vi "HFRR ADV v038.vi"() -> ()   [LabVIEW 2025] (continued)
        n1305 = case shown="True" w1608 {
          selector: w1608 -> [_ w1614]
          frame False {
          }
          frame True {
            n1306 = Not(x=w1614) -> (.not. x?=w1613:bool)
            n1307 = local write "CAMERA ROI MIN TEMP"(w1613) -> ()
            n1308 = call "IMAGE ANALYSIS.vi"("Enum"=POST_ANALYSIS_ENUM."MINIMIZE UI") -> ()  [unwired: 9 in, 2 out]
          }
        }
      }
      frame "Mooha" {
        n1309 = local read "LIVE FEED MIN TEMP"() -> (w1620:bool)
        n1310 = local write "LIVE FEED MAX TEMP"(TRUE ("LIVE FEED MAX TEMP")) -> ()
        n1311 = local read "CAMERA ROI MIN TEMP"() -> (w1618:bool)
        n1312 = case shown="True" w1620 {
          selector: w1620 -> [_ w1627]
          frame False {
          }
          frame True {
            n1313 = Not(x=w1627) -> (.not. x?=w1626:bool)
            n1314 = local write "LIVE FEED MIN TEMP"(w1626) -> ()
            n1315 = call "CAMERA LIVE FEED FGV.vi"("Enum - Menu"=CAMERA_LIVE_FEED_ENUM."CAMERA MINIMIZE") -> ()  [unwired: 9 in, 2 out]
          }
        }
        n1316 = local write "CAMERA ROI MAX TEMP"(TRUE ("CAMERA ROI MAX TEMP")) -> ()
        n1317 = case shown="True" w1618 {
          selector: w1618 -> [_ w1624]
          frame False {
          }
          frame True {
            n1318 = Not(x=w1624) -> (.not. x?=w1623:bool)
            n1319 = local write "CAMERA ROI MIN TEMP"(w1623) -> ()
            n1320 = call "IMAGE ANALYSIS.vi"("Enum"=POST_ANALYSIS_ENUM."MINIMIZE UI") -> ()  [unwired: 9 in, 2 out]
          }
        }
      }
    }
    n1321 = local read "Auto Start Test"() -> (w1365:bool)
    n1322 = case shown="True" "sign in temp" {
      frame False {
      }
      frame True {
        w1400 = 1 ("y")
        n1323 = local read "USERNAME"() -> (w1406:string)
        n1324 = local read "USER ID"() -> (w1403:string)
        n1325 = call <vilib>:"Trim Whitespace.vi"("string"=w1406) -> ("trimmed string"=w1405:string)  [unwired: 1 in]
        n1326 = call <vilib>:"Trim Whitespace.vi"("string"=w1403) -> ("trimmed string"=w1404:string)  [unwired: 1 in]
        n1327 = String Length(string=w1405) -> (length=w1402:i32)
        n1328 = String Length(string=w1404) -> (length=w1401:i32)
        n1329 = Greater?(x=w1402, y=w1400) -> (0:w1399:bool)
        n1330 = Greater?(x=w1401, y=w1400) -> (0:w1398:bool)
        n1331 = And(x=w1399, y=w1398) -> (x .and. y?=w1397:bool)
        n1332 = case shown="True" w1397 {
          frame False {
            n1333 = property on="Sign In" class="Bool (strict)"("DisabledEnum"=T19."Disabled" ("Disabled")) -> ()  [unwired: 2 in, 2 out]
          }
          frame True {
            n1334 = property on="Sign In" class="Bool (strict)"("DisabledEnum"=T19."Enabled" ("Disabled")) -> ()  [unwired: 2 in, 2 out]
          }
        }
      }
    }
    n1335 = local read "Air Temperature"() -> (w1382:bool)
    n1336 = local read "Coefficient Of Friction"() -> (w1383:bool)
    n1337 = case shown="False" w1365 {
      frame False {
        n1338 = local read "Auto stop temp"() -> (w1394:bool)
        n1339 = case shown="True" w1394 {
          frame False {
          }
          frame True {
            n1340 = local write "Auto Start Temp"(FALSE ("Auto Start Temp")) -> ()
          }
        }
      }
      frame True {
        "Auto stop temp" <- TRUE ("Auto stop temp")
      }
    }
    n1341 = local read "Humidity"() -> (w1381:bool)
    n1342 = case shown="\"HOME\"" w1391 {
      frame "HOME" {
        n1343 = local write "main tab sub"(enum32{"Page 1", "Page 2"}."Page 1" ("main tab sub")) -> ()
      }
      frame Default {
        n1344 = local write "main tab sub"(enum32{"Page 1", "Page 2"}."Page 2" ("main tab sub")) -> ()
      }
    }
    n1345 = case shown="True" w1390 {
      selector: w1390 -> [_ w1742]
      frame False {
      }
      frame True {
        n1346 = Not(x=w1742) -> (.not. x?=w1741:bool)
        n1347 = local write "Sign In"(w1741) -> ()
        n1348 = local write "Main Dashboard Buttons"(T26."Test Setup" ("Main Dashboard Buttons")) -> ()
      }
    }
    n1349 = case shown="\"Numeric Display\", Default" "Num/Graph" {
      frame "Numeric Display", Default {
        n1350 = property on="Single/Multiple" class="RadioBtnsControl (strict)"("Visible"=FALSE) -> ()  [unwired: 2 in, 2 out]
        n1351 = property on="Single - Graph" class="Ring (strict)"("Visible"=FALSE) -> ()  [unwired: 2 in, 2 out]
        n1352 = local write "Main Tab Display"(T4."Dashboard 1" ("Main Tab Display")) -> ()
      }
      frame "Graph Display" {
        n1353 = property on="Single/Multiple" class="RadioBtnsControl (strict)"("Visible"=TRUE) -> ()  [unwired: 2 in, 2 out]
        n1354 = case shown="\"Multiple\"" "Single/Multiple" {
          frame "Single ", Default {
            n1355 = property on="Single - Graph" class="Ring (strict)"("Visible"=TRUE) -> ()  [unwired: 2 in, 2 out]
            n1356 = local write "Main Tab Display"(T4."Dashboard 3" ("Main Tab Display")) -> ()
          }
          frame "Multiple" {
            n1357 = property on="Single - Graph" class="Ring (strict)"("Visible"=FALSE) -> ()  [unwired: 2 in, 2 out]
            n1358 = local write "Main Tab Display"(T4."Dashboard 2" ("Main Tab Display")) -> ()
          }
        }
      }
    }
    n1359 = local read "Stroke"() -> (w1380:bool)
    n1360 = local read "USERNAME"() -> (w1385:string)
    n1361 = case shown="True" w1383 {
      selector: w1383 -> [_ w1667]
      frame False {
      }
      frame True {
        n1362 = Not(x=w1667) -> (.not. x?=w1666:bool)
        n1363 = local write "Coefficient Of Friction"(w1666) -> ()
        n1364 = local write "Tab Control 2"(T6."Coefficient Of Friction" ("Tab Control 2")) -> ()
      }
    }
    n1365 = case shown="True" w1382 {
      selector: w1382 -> [_ w1664]
      frame False {
      }
      frame True {
        n1366 = Not(x=w1664) -> (.not. x?=w1662:bool)
        n1367 = local write "Air Temperature"(w1662) -> ()
        n1368 = local write "Tab Control 2"(T6."Air Temperature" ("Tab Control 2")) -> ()
      }
    }
    n1369 = case shown="True" w1380 {
      selector: w1380 -> [_ w1658]
      frame False {
      }
      frame True {
        n1370 = Not(x=w1658) -> (.not. x?=w1656:bool)
        n1371 = local write "Stroke"(w1656) -> ()
        n1372 = local write "Tab Control 2"(T6."Stroke" ("Tab Control 2")) -> ()
      }
    }
    n1373 = local write "tested by"(w1385) -> ()
    n1374 = case shown="True" w1381 {
      selector: w1381 -> [_ w1661]
      frame False {
      }
      frame True {
        n1375 = Not(x=w1661) -> (.not. x?=w1659:bool)
        n1376 = local write "Humidity"(w1659) -> ()
        n1377 = local write "Tab Control 2"(T6."Humidity" ("Tab Control 2")) -> ()
      }
    }
    n1378 = case shown="\"Calibration\"" "Main Dashboard Buttons" {
      tunnel: [T2."HOME" ("Main Tab") T2."Test Setup" ("Main Tab") T2."Acquire" ("Main Tab") T2."Adv Scar" ("Main Tab") T2."Adv Scar Report" ("Main Tab") T2."Compare Files" ("Main Tab") T2."Calibration" ("Main Tab") T2."About" ("Main Tab") T2."Advance" ("Main Tab")] -> w1364
      frame "Home", Default {
      }
      frame "Test Setup" {
      }
      frame "Dashboard" {
      }
      frame "Imaging" {
      }
      frame "Report" {
      }
      frame "Analysis" {
      }
      frame "Calibration" {
      }
      frame "About" {
      }
      frame "Advance" {
      }
    }
    n1379 = Wait (ms)(milliseconds to wait=u32 100) -> ()  [unwired: 1 out]
    n1380 = local read "Main Tab Display"() -> (w1384:T4)
    n1381 = local write "Main Tab"(w1364) -> ()
    n1382 = case shown="\"Dashboard 3\"" w1384 {
      frame "Dashboard 1", Default {
        n1383 = property on="Reset Graph" class="Bool (strict)"("Visible"=FALSE) -> ()  [unwired: 2 in, 2 out]
      }
      frame "Dashboard 2" {
        n1384 = property on="Reset Graph" class="Bool (strict)"("Visible"=TRUE) -> ()  [unwired: 2 in, 2 out]
      }
      frame "Dashboard 3" {
        n1385 = property on="Reset Graph" class="Bool (strict)"("Visible"=TRUE) -> ()  [unwired: 2 in, 2 out]
      }
    }
    n1386 = local read "SCAR MEASURMENT"() -> (w1372:enum32{"Auto Scar", "Manual Scar"})
    n1387 = local read "Humidity"() -> (w1386:bool)
    n1388 = local read "Cap Live Image"() -> (w1369:bool)
    n1389 = local read "Sample Temperature"() -> (w1379:bool)
    n1390 = local read "Air Temp vs Humidity"() -> (w1377:bool)
    n1391 = local read "Frequency"() -> (w1378:bool)
    n1392 = case shown="False" w1386 {
      frame False {
        n1393 = local write "Humidity On Command"(TRUE ("Humidity On Command")) -> ()
        n1394 = case shown="True" "Humidity Off Command" {
          selector: "Humidity Off Command" -> [_ w1674]
          frame False {
          }
          frame True {
            n1395 = stacked-sequence {
              frame #0 {
                n1396 = local read "WriteHumidity"() -> (w1676:string[])
                n1397 = Insert Into Array(array=w1676, new element="R;1" ("new element/subarray")) -> (w1675:string[])  [unwired: 1 in]
                n1398 = local write "WriteHumidity"(w1675) -> ()
              }
              frame #1 {
                n1399 = Wait (ms)(milliseconds to wait=u32 500) -> ()  [unwired: 1 out]
              }
              frame #2 {
                n1400 = local read "WriteHumidity"() -> (w1680:string[])
                n1401 = local read "EVENT LOG"() -> (w1684:string)
                n1402 = call "Event Log.vi"("Content"="Humidity Control Off" ("string"), "EVENT LOG"=w1684) -> ("EVENT LOG"=w1685:string)  [unwired: 8 in, 1 out]
                n1403 = local write "EVENT LOG"(w1685) -> ()
                n1404 = Insert Into Array(array=w1680, new element="R;1" ("new element/subarray")) -> (w1681:string[])  [unwired: 1 in]
                n1405 = local write "WriteHumidity"(w1681) -> ()
                n1406 = local write "Humidity"(TRUE ("Humidity")) -> ()
              }
            }
            n1407 = Not(x=w1674) -> (.not. x?=w1673:bool)
            n1408 = local write "Humidity Off Command"(w1673) -> ()
          }
        }
      }
      frame True {
        n1409 = local write "Humidity Off Command"(TRUE ("Humidity Off Command")) -> ()
        n1410 = case shown="False" "Humidity On Command" {
          selector: "Humidity On Command" -> [_ w1689]
          frame False {
          }
          frame True {
            n1411 = stacked-sequence {
              frame #0 {
                n1412 = local read "Set Rh"() -> (w1695:dbl)
                n1413 = local read "WriteHumidity"() -> (w1691:string[])
                n1414 = Number To Fractional String(number=w1695, precision (6)=i16 2) -> (F-format string=w1696:string)  [unwired: 2 in]
                n1415 = Concatenate Strings("M;" ("new element/subarray"), w1696) -> (w1694:string)
                n1416 = Insert Into Array(array=w1691, new element=w1694) -> (w1690:string[])  [unwired: 1 in]
                n1417 = local write "WriteHumidity"(w1690) -> ()
              }
              frame #1 {
                n1418 = Wait (ms)(milliseconds to wait=u32 500) -> ()  [unwired: 1 out]
              }
              frame #2 {
                n1419 = local read "WriteHumidity"() -> (w1699:string[])
                n1420 = local read "Set Rh"() -> (w1703:dbl)
                n1421 = Number To Fractional String(number=w1703, precision (6)=i16 2) -> (F-format string=w1704:string)  [unwired: 2 in]
                n1422 = Concatenate Strings("M;" ("new element/subarray"), w1704) -> (w1702:string)
                n1423 = Insert Into Array(array=w1699, new element=w1702) -> (w1698:string[])  [unwired: 1 in]
                n1424 = local write "WriteHumidity"(w1698) -> ()
              }
              frame #3 {
                n1425 = Wait (ms)(milliseconds to wait=u32 500) -> ()  [unwired: 1 out]
              }
              frame #4 {
                (unwired) "% RH" ("string")
                (unwired) i16 2 ("precision (6)")
                (unwired) "M;" ("new element/subarray")
                n1426 = local read "Set Rh"() -> (w1713:dbl)
                n1427 = local read "WriteHumidity"() -> (w1706:string[])
                n1428 = Number To Fractional String(number=w1713, precision (6)=i16 2) -> (F-format string=w1710:string)  [unwired: 2 in]
                n1429 = Concatenate Strings("M;" ("new element/subarray"), w1710) -> (w1714:string)
                n1430 = Concatenate Strings("Humidity Set to : " ("string"), w1710, "% RH" ("string")) -> (w1708:string)
                n1431 = Insert Into Array(array=w1706, new element=w1714) -> (w1707:string[])  [unwired: 1 in]
                n1432 = disable-structure shown="Enabled" {
                  frame Enabled {
                    n1433 = local read "EVENT LOG"() -> (w1717:string)
                    n1434 = call "Event Log.vi"("Content"="Humidity Control On", "EVENT LOG"=w1717) -> ("EVENT LOG"=w1718:string)  [unwired: 8 in, 1 out]
                    n1435 = local write "EVENT LOG"(w1718) -> ()
                  }
                  frame Disabled {
                  }
                }
                n1436 = disable-structure shown="Enabled" {
                  disable-tunnel: w1708 -> [_ _]
                  frame Enabled {
                    n1437 = local read "EVENT LOG"() -> (w1720:string)
                    n1438 = call "Event Log.vi"("Content"="Humidity Control On", "EVENT LOG"=w1720) -> ("EVENT LOG"=w1721:string)  [unwired: 8 in, 1 out]
                    n1439 = local write "EVENT LOG"(w1721) -> ()
                  }
                  frame Disabled {
                  }
                }
                n1440 = local write "WriteHumidity"(w1707) -> ()
              }
            }
            n1441 = Not(x=w1689) -> (.not. x?=w1688:bool)
            n1442 = local write "Humidity On Command"(w1688) -> ()
          }
        }
      }
    }
    n1443 = Equal?(x=w1372, y=enum32{"Auto Scar", "Manual Scar"}."Auto Scar" ("SCAR MEASURMENT")) -> (x = y?=w1368:bool)
    n1444 = local read "TEST STANDARD"() -> (w1375:T3)
    n1445 = And(x=w1369, y=w1368) -> (x .and. y?=w1370:bool)
    n1446 = case shown="True" w1370 {
      selector: w1370 -> [_ w1473]
      tunnel: errorcluster {"status"=FALSE, "code"=0, "source"=""} ("error in (no error) 3") -> [_ w1474]
      frame False {
      }
      frame True {
        n1447 = stacked-sequence {
          tunnel: w1474 -> [_ _ _ _ _ _ _ w1522]
          tunnel: w1473 -> [_ _ _ _ _ w1503 _ _]
          frame #0 {
            n1448 = call "CAMERA LIVE FEED FGV.vi"("Enum - Menu"=CAMERA_LIVE_FEED_ENUM."CAMERA MINIMIZE") -> ()  [unwired: 9 in, 2 out]
          }
          frame #1 {
            n1449 = property on="Auto Scar Check  2" class="Clust (strict)"("Visible"=TRUE) -> ()  [unwired: 2 in, 2 out]
          }
          frame #2 {
            n1450 = String To Path(string="C:\\LAB-IQ\\Image Calibrate v01.dcf") -> (path=w1479:path)
            n1451 = Open/Create/Replace File ("Open File")(file path (use dialog)=w1479) -> (refnum out=w1480:refnum<file>)  [unwired: 5 in, 2 out]
            n1452 = for {
              N: 4 -> [_]
              tunnel: w1480 -> [w1486]
              i -> [w1482]
              n1453 = Read from Text File ("Read File")(file (use dialog)=w1486) -> (text=w1487:string)  [unwired: 3 in, 3 out]
              n1454 = String Subset(string=w1487, offset (0)=6, length (rest)=10 ("length (rest)")) -> (substring=w1483:string)
              n1455 = Fract/Exp String To Number(string=w1483) -> (number=w1481:dbl)  [unwired: 3 in, 1 out]
              n1456 = case shown="0" w1482 {
                tunnel: w1481 -> [w1488 w1489 _ w1490 _]
                frame 0 {
                  "5x Gain" <- w1488
                }
                frame 1 {
                  "10x Gain" <- w1489
                }
                frame 2 {
                }
                frame 3 {
                  "100x gain" <- w1490
                }
                frame 4, Default {
                }
              }
            }
          }
          frame #3 {
            n1457 = local read "FILE 3"() -> (w1496:string)
            n1458 = call <vilib>:"Trim Whitespace.vi"("string"="C:\\LAB-IQ\\images\\") -> ("trimmed string"=w1498:string)  [unwired: 1 in]
            n1459 = String To Path(string=w1498) -> (path=w1497:path)
            n1460 = Concatenate Strings(w1496, ".png" ("string")) -> (w1495:string)
            n1461 = Build Path(base path=w1497, name or relative path=w1495) -> (appended path=w1493:path)
            "Image path" <- w1493
            n1462 = Path To String(path=w1493) -> (string=w1492:string)
            n1463 = call "CAMERA LIVE FEED FGV.vi"("Enum - Menu"=CAMERA_LIVE_FEED_ENUM."CAMERA SAVE", "Image Path"=w1492) -> ()  [unwired: 8 in, 2 out]
          }
          frame #4 {
            n1464 = One Button Dialog(message="Image saved successfully") -> ()  [unwired: 1 in, 1 out]
          }
          frame #5 {
            n1465 = local read "TEST STANDARD"() -> (w1502:T3)
            n1466 = local read "Magnification len live scar"() -> (w1514:string)
            n1467 = Not(x=w1503) -> (.not. x?=w1504:bool)
            n1468 = local write "Cap Live Image"(w1504) -> ()
            n1469 = case shown="\"ISO 12156\"" w1502 {
              tunnel: ["ASTM D6079" "ISO 12156"] -> w1501
              frame "ASTM D6079", Default {
              }
              frame "ISO 12156" {
              }
            }
            n1470 = case shown="\"5x\", Default" w1514 {
              tunnel: [w1517 w1518] -> w1513
              frame "5x", Default {
                n1471 = local read "5x Gain"() -> (w1517:dbl)
              }
              frame "10x" {
                # "5x"
                n1472 = local read "10x Gain"() -> (w1518:dbl)
              }
            }
            n1473 = local read "Image path"() -> (w1512:path)
            n1474 = local read "FILE 3"() -> (w1505:string)
            n1475 = call "EDGE DETCTION.vi"("GAIN VALUE"=w1513, "Image Path"=w1512) -> ("error out"=w1511:errorcluster, "return value"=w1510:cluster{string, string, dbl, dbl, dbl})  [unwired: 8 in]
            n1476 = Bundle By Name(cluster=T27 {"File Name"="", "Test Method"="", "Operator"="", "Fuel Description"="", "Date and time"=""} ("Main Ref"), "File Name"=w1505, "Test Method"=w1501) -> (w1506:T27)
            n1477 = call "duf file read.vi"("error in (no error)"=w1511, "Main Ref"=w1506) -> ("error out"=w1509:errorcluster, "Main Ref 2"=w1507:T27)  [unwired: 8 in]
            n1478 = call "EDGE DETECTION REPORT.vi"("error in (no error)"=w1509, "return value 2"=w1510, "Main Ref"=w1507) -> ()  [unwired: 8 in, 1 out]
          }
          frame #6 {
            n1479 = property on="Auto Scar Check  2" class="Clust (strict)"("Visible"=FALSE) -> ()  [unwired: 2 in, 2 out]
          }
          frame #7 {
            n1480 = call "CAMERA LIVE FEED FGV.vi"("Enum - Menu"=CAMERA_LIVE_FEED_ENUM."CAMERA MINIMIZE", "error in (no error)"=w1522) -> ()  [unwired: 8 in, 2 out]
            n1481 = local write "Main Dashboard Buttons"(T1."Home" ("Main Dashboard Buttons")) -> ()
            n1482 = local write "Main Tab"(T2."HOME" ("Main Tab")) -> ()
          }
        }
      }
    }
    n1483 = local read "Heater Button"() -> (w1376:bool)
    n1484 = case shown="True" w1378 {
      selector: w1378 -> [_ w1652]
      frame False {
      }
      frame True {
        n1485 = Not(x=w1652) -> (.not. x?=w1650:bool)
        n1486 = local write "Frequency"(w1650) -> ()
        n1487 = local write "Tab Control 2"(T6."Frequency" ("Tab Control 2")) -> ()
      }
    }
    n1488 = case shown="True" w1377 {
      selector: w1377 -> [_ w1649]
      frame False {
      }
      frame True {
        n1489 = Not(x=w1649) -> (.not. x?=w1647:bool)
        n1490 = local write "Air Temp vs Humidity"(w1647) -> ()
        n1491 = local write "Tab Control 2"(T6."Air Temp vs Rh" ("Tab Control 2")) -> ()
      }
    }
    n1492 = case shown="True" w1379 {
      selector: w1379 -> [_ w1655]
      frame False {
      }
      frame True {
        n1493 = Not(x=w1655) -> (.not. x?=w1653:bool)
        n1494 = local write "Sample Temperature"(w1653) -> ()
        n1495 = local write "Tab Control 2"(T6."Sample Temperature" ("Tab Control 2")) -> ()
      }
    }
    n1496 = case shown="\"Custom\"" w1375 {
      frame "ASTM D6079", Default {
        w1628 = "ASTM D6079 TEST CONDITIONS" ("Standard 2")
        n1497 = local write "Standard 2"(w1628) -> ()
        n1498 = local write "Standard"(w1628) -> ()
      }
      frame "ISO 12156" {
        w1629 = "ISO 12156 TEST CONDITIONS" ("Standard 2")
        n1499 = local write "Standard 2"(w1629) -> ()
        n1500 = local write "Standard"(w1629) -> ()
      }
      frame "CEC F-096-A-06" {
        w1630 = "CEC F-096-A-06 TEST CONDITIONS" ("Standard 2")
        n1501 = local write "Standard 2"(w1630) -> ()
        n1502 = local write "Standard"(w1630) -> ()
      }
      frame "Custom" {
        w1631 = "CUSTOM TEST CONDITIONS" ("Standard 2")
        n1503 = local write "Standard 2"(w1631) -> ()
        n1504 = local write "Standard"(w1631) -> ()
      }
    }
    n1505 = case shown="True" w1376 {
      frame False {
        n1506 = local write "Temperature On Command"(TRUE ("Temperature On Command")) -> ()
        n1507 = case shown="True" "Temperature Off Command" {
          selector: "Temperature Off Command" -> [_ w1635]
          frame False {
          }
          frame True {
            n1508 = Not(x=w1635) -> (.not. x?=w1634:bool)
            n1509 = local read "EVENT LOG"() -> (w1638:string)
            n1510 = local write "Temperature Off Command"(w1634) -> ()
            n1511 = call "Event Log.vi"("Content"="Heater Off", "EVENT LOG"=w1638) -> ("EVENT LOG"=w1637:string)  [unwired: 8 in, 1 out]
            n1512 = local write "EVENT LOG"(w1637) -> ()
          }
        }
      }
      frame True {
        n1513 = local write "Temperature Off Command"(TRUE ("Temperature Off Command")) -> ()
        n1514 = case shown="True" "Temperature On Command" {
          selector: "Temperature On Command" -> [_ w1642]
          frame False {
          }
          frame True {
            n1515 = Not(x=w1642) -> (.not. x?=w1641:bool)
            n1516 = local write "Temperature On Command"(w1641) -> ()
            n1517 = disable-structure shown="Enabled" {
              disable-tunnel: "Heater On" -> [w1644 _]
              frame Enabled {
                n1518 = local read "EVENT LOG"() -> (w1645:string)
                n1519 = call "Event Log.vi"("Content"=w1644, "EVENT LOG"=w1645) -> ("EVENT LOG"=w1646:string)  [unwired: 8 in, 1 out]
                n1520 = local write "EVENT LOG"(w1646) -> ()
              }
              frame Disabled {
              }
            }
          }
        }
      }
    }
    n1521 = local read "Main Tab"() -> (w1367:T2)
    n1522 = case shown="\"About\"" w1367 {
      frame "HOME", Default {
        w1409 = T19."Enabled" ("Disabled")
        n1523 = local read "Service Password enable"() -> (w1411:bool)
        n1524 = property on="Imaging" class="Bool (strict)"("DisabledEnum"=w1409) -> ()  [unwired: 2 in, 2 out]
        n1525 = property on="Dashboard" class="Bool (strict)"("DisabledEnum"=w1409) -> ()  [unwired: 2 in, 2 out]
        n1526 = property on="Test Setup" class="Bool (strict)"("DisabledEnum"=w1409) -> ()  [unwired: 2 in, 2 out]
        n1527 = property on="Analysis" class="Bool (strict)"("DisabledEnum"=w1409) -> ()  [unwired: 2 in, 2 out]
        n1528 = property on="Home" class="Bool (strict)"("DisabledEnum"=w1409) -> ()  [unwired: 2 in, 2 out]
        n1529 = property on="Report" class="Bool (strict)"("DisabledEnum"=w1409) -> ()  [unwired: 2 in, 2 out]
        n1530 = property on="Main Dashboard Buttons" class="RadioBtnsControl (strict)"("DisabledEnum"=w1409) -> ()  [unwired: 2 in, 2 out]
        n1531 = property on="Calibration" class="Bool (strict)"("DisabledEnum"=w1409) -> ()  [unwired: 2 in, 2 out]
        n1532 = case shown="True" w1411 {
          tunnel: [T19."Disabled" ("Disabled") T19."Enabled" ("Disabled")] -> w1410
          frame False {
          }
          frame True {
          }
        }
        n1533 = property on="About" class="Bool (strict)"("DisabledEnum"=w1410) -> ()  [unwired: 2 in, 2 out]
      }
      frame "Test Setup" {
        w1416 = T19."Enabled" ("Disabled")
        n1534 = local read "Service Password enable"() -> (w1415:bool)
        n1535 = property on="Dashboard" class="Bool (strict)"("DisabledEnum"=T19."Disabled" ("Disabled")) -> ()  [unwired: 2 in, 2 out]
        n1536 = property on="Imaging" class="Bool (strict)"("DisabledEnum"=w1416) -> ()  [unwired: 2 in, 2 out]
        n1537 = property on="Analysis" class="Bool (strict)"("DisabledEnum"=w1416) -> ()  [unwired: 2 in, 2 out]
        n1538 = property on="Home" class="Bool (strict)"("DisabledEnum"=w1416) -> ()  [unwired: 2 in, 2 out]
        n1539 = property on="Report" class="Bool (strict)"("DisabledEnum"=w1416) -> ()  [unwired: 2 in, 2 out]
        n1540 = property on="Test Setup" class="Bool (strict)"("DisabledEnum"=w1416) -> ()  [unwired: 2 in, 2 out]
        n1541 = case shown="True" w1415 {
          tunnel: [T19."Disabled" ("Disabled") T19."Enabled" ("Disabled")] -> w1414
          frame False {
          }
          frame True {
          }
        }
        n1542 = property on="About" class="Bool (strict)"("DisabledEnum"=w1414) -> ()  [unwired: 2 in, 2 out]
      }
      frame "Adv Scar" {
        w1423 = T19."Enabled" ("Disabled")
        n1543 = property on="Dashboard" class="Bool (strict)"("DisabledEnum"=T19."Disabled" ("Disabled")) -> ()  [unwired: 2 in, 2 out]
        n1544 = property on="Imaging" class="Bool (strict)"("DisabledEnum"=w1423) -> ()  [unwired: 2 in, 2 out]
        n1545 = property on="Analysis" class="Bool (strict)"("DisabledEnum"=w1423) -> ()  [unwired: 2 in, 2 out]
        n1546 = property on="Home" class="Bool (strict)"("DisabledEnum"=w1423) -> ()  [unwired: 2 in, 2 out]
        n1547 = property on="Report" class="Bool (strict)"("DisabledEnum"=w1423) -> ()  [unwired: 2 in, 2 out]
        n1548 = property on="Test Setup" class="Bool (strict)"("DisabledEnum"=w1423) -> ()  [unwired: 2 in, 2 out]
        n1549 = local read "Service Password enable"() -> (w1421:bool)
        n1550 = case shown="True" w1421 {
          tunnel: [T19."Disabled" ("Disabled") T19."Enabled" ("Disabled")] -> w1420
          frame False {
          }
          frame True {
          }
        }
        n1551 = property on="About" class="Bool (strict)"("DisabledEnum"=w1420) -> ()  [unwired: 2 in, 2 out]
      }
      frame "Calibration" {
        w1426 = T19."Enabled" ("Disabled")
        n1552 = property on="Dashboard" class="Bool (strict)"("DisabledEnum"=T19."Disabled" ("Disabled")) -> ()  [unwired: 2 in, 2 out]
        n1553 = property on="Imaging" class="Bool (strict)"("DisabledEnum"=w1426) -> ()  [unwired: 2 in, 2 out]
        n1554 = property on="Analysis" class="Bool (strict)"("DisabledEnum"=w1426) -> ()  [unwired: 2 in, 2 out]
        n1555 = property on="Home" class="Bool (strict)"("DisabledEnum"=w1426) -> ()  [unwired: 2 in, 2 out]
        n1556 = property on="Report" class="Bool (strict)"("DisabledEnum"=w1426) -> ()  [unwired: 2 in, 2 out]
        n1557 = property on="Test Setup" class="Bool (strict)"("DisabledEnum"=w1426) -> ()  [unwired: 2 in, 2 out]
        n1558 = local read "Service Password enable"() -> (w1428:bool)
        n1559 = property on="Calibration" class="Bool (strict)"("DisabledEnum"=w1426) -> ()  [unwired: 2 in, 2 out]
        n1560 = case shown="True" w1428 {
          tunnel: [T19."Disabled" ("Disabled") T19."Enabled" ("Disabled")] -> w1427
          frame False {
          }
          frame True {
          }
        }
        n1561 = property on="About" class="Bool (strict)"("DisabledEnum"=w1427) -> ()  [unwired: 2 in, 2 out]
      }
      frame "Adv Scar Report" {
        w1434 = T19."Enabled" ("Disabled")
        n1562 = property on="Dashboard" class="Bool (strict)"("DisabledEnum"=T19."Disabled" ("Disabled")) -> ()  [unwired: 2 in, 2 out]
        n1563 = property on="Imaging" class="Bool (strict)"("DisabledEnum"=w1434) -> ()  [unwired: 2 in, 2 out]
        n1564 = property on="Analysis" class="Bool (strict)"("DisabledEnum"=w1434) -> ()  [unwired: 2 in, 2 out]
        n1565 = property on="Home" class="Bool (strict)"("DisabledEnum"=w1434) -> ()  [unwired: 2 in, 2 out]
        n1566 = property on="Report" class="Bool (strict)"("DisabledEnum"=w1434) -> ()  [unwired: 2 in, 2 out]
        n1567 = property on="Test Setup" class="Bool (strict)"("DisabledEnum"=w1434) -> ()  [unwired: 2 in, 2 out]
        n1568 = local read "Service Password enable"() -> (w1433:bool)
        n1569 = case shown="True" w1433 {
          tunnel: [T19."Disabled" ("Disabled") T19."Enabled" ("Disabled")] -> w1432
          frame False {
          }
          frame True {
          }
        }
        n1570 = property on="About" class="Bool (strict)"("DisabledEnum"=w1432) -> ()  [unwired: 2 in, 2 out]
      }
      frame "Compare Files" {
        w1440 = T19."Enabled" ("Disabled")
        n1571 = local read "Service Password enable"() -> (w1439:bool)
        n1572 = property on="Dashboard" class="Bool (strict)"("DisabledEnum"=T19."Disabled" ("Disabled")) -> ()  [unwired: 2 in, 2 out]
        n1573 = property on="Imaging" class="Bool (strict)"("DisabledEnum"=w1440) -> ()  [unwired: 2 in, 2 out]
        n1574 = property on="Analysis" class="Bool (strict)"("DisabledEnum"=w1440) -> ()  [unwired: 2 in, 2 out]
        n1575 = property on="Home" class="Bool (strict)"("DisabledEnum"=w1440) -> ()  [unwired: 2 in, 2 out]
        n1576 = property on="Report" class="Bool (strict)"("DisabledEnum"=w1440) -> ()  [unwired: 2 in, 2 out]
        n1577 = property on="Test Setup" class="Bool (strict)"("DisabledEnum"=w1440) -> ()  [unwired: 2 in, 2 out]
        n1578 = case shown="True" w1439 {
          tunnel: [T19."Disabled" ("Disabled") T19."Enabled" ("Disabled")] -> w1438
          frame False {
          }
          frame True {
          }
        }
        n1579 = property on="About" class="Bool (strict)"("DisabledEnum"=w1438) -> ()  [unwired: 2 in, 2 out]
      }
      frame "Acquire" {
        n1580 = local read "Service Password enable"() -> (w1445:bool)
        n1581 = property on="Test Setup" class="Bool (strict)"("DisabledEnum"=T19."Disabled" ("Disabled")) -> ()  [unwired: 2 in, 2 out]
        n1582 = local read "Auto Start Test"() -> (w1447:bool)
        n1583 = local read "RUN"() -> (w1449:bool)
        n1584 = case shown="True" w1445 {
          tunnel: [T19."Disabled" ("Disabled") T19."Enabled" ("Disabled")] -> w1446
          frame False {
          }
          frame True {
          }
        }
        n1585 = Or(x=w1449, y=w1447) -> (x .or. y?=w1448:bool)
        n1586 = case shown="True" w1448 {
          tunnel: [T19."Enabled" ("Disabled") T19."Disabled" ("Disabled")] -> w1444
          frame False {
          }
          frame True {
          }
        }
        n1587 = property on="About" class="Bool (strict)"("DisabledEnum"=w1446) -> ()  [unwired: 2 in, 2 out]
        n1588 = property on="Imaging" class="Bool (strict)"("DisabledEnum"=w1444) -> ()  [unwired: 2 in, 2 out]
        n1589 = property on="Dashboard" class="Bool (strict)"("DisabledEnum"=w1444) -> ()  [unwired: 2 in, 2 out]
        n1590 = property on="Analysis" class="Bool (strict)"("DisabledEnum"=w1444) -> ()  [unwired: 2 in, 2 out]
        n1591 = property on="Home" class="Bool (strict)"("DisabledEnum"=w1444) -> ()  [unwired: 2 in, 2 out]
        n1592 = property on="Report" class="Bool (strict)"("DisabledEnum"=w1444) -> ()  [unwired: 2 in, 2 out]
        n1593 = property on="Calibration" class="Bool (strict)"("DisabledEnum"=w1444) -> ()  [unwired: 2 in, 2 out]
      }
      frame "About" {
        n1594 = local read "FILE"() -> (w1463:string)
        n1595 = local read "TEST FILE NAM,E SAVED"() -> (w1456:bool)
        n1596 = call <vilib>:"Trim Whitespace.vi"("string"=w1463) -> ("trimmed string"=w1462:string)  [unwired: 1 in]
        n1597 = local read "Auto Start Test"() -> (w1466:bool)
        n1598 = String Length(string=w1462) -> (length=w1461:i32)
        n1599 = Greater?(x=w1461, y=1) -> (0:w1458:bool)
        n1600 = And(x=w1458, y=w1456) -> (x .and. y?=w1457:bool)
        n1601 = local read "RUN"() -> (w1468:bool)
        n1602 = case shown="True" w1457 {
          tunnel: [T19."Disabled" ("Disabled") T19."Enabled" ("Disabled")] -> w1459
          frame False {
          }
          frame True {
          }
        }
        n1603 = Or(x=w1468, y=w1466) -> (x .or. y?=w1467:bool)
        n1604 = property on="About" class="Bool (strict)"("DisabledEnum"=T19."Enabled" ("Disabled")) -> ()  [unwired: 2 in, 2 out]
        n1605 = case shown="False" w1467 {
          tunnel: [T19."Enabled" ("Disabled") T19."Disabled" ("Disabled")] -> w1465
          frame False {
          }
          frame True {
          }
        }
        n1606 = property on="Dashboard" class="Bool (strict)"("DisabledEnum"=w1459) -> ()  [unwired: 2 in, 2 out]
        n1607 = property on="Test Setup" class="Bool (strict)"("DisabledEnum"=T19."Disabled" ("Disabled")) -> ()  [unwired: 2 in, 2 out]
        n1608 = property on="Imaging" class="Bool (strict)"("DisabledEnum"=w1465) -> ()  [unwired: 2 in, 2 out]
        n1609 = property on="Analysis" class="Bool (strict)"("DisabledEnum"=w1465) -> ()  [unwired: 2 in, 2 out]
        n1610 = property on="Home" class="Bool (strict)"("DisabledEnum"=w1465) -> ()  [unwired: 2 in, 2 out]
        n1611 = property on="Report" class="Bool (strict)"("DisabledEnum"=w1465) -> ()  [unwired: 2 in, 2 out]
      }
    }
    n1612 = local read "Quit"() -> (w1393:bool)
    "Single" <- "Single - Graph"
  }
  n1613 = disable-structure shown="Disabled" {
    disable-tunnel: [w1746 _] -> w42
    disable-tunnel: _ -> [w1745 _]
    frame Disabled {
      n1614 = while {
        tunnel: w1745 -> [_]
        tunnel: [w1747] -> w1746
        tunnel: [w1748] -> _
        i -> [w1748]
        stop <- w1747 stop-if-true
        w1764 = u16 10 items=["1.0"=10, "1.5"=15, "2.0"=20] ("stop bits (10: 1 bit)")
        n1615 = Wait (ms)(milliseconds to wait=u32 10) -> ()  [unwired: 1 out]
        n1616 = call-poly "VISA Configure Serial Port"("VISA resource name"=refnum<visa-resource-name> "ASRL1::INSTR" ("COM PORT"), "timeout (10sec)"=u32 10, "baud rate (9600)"=u32 57600, "data bits (8)"=u16 8, "stop bits (10: 1 bit)"=w1764) -> ("VISA resource name out"=w1750:refnum<visa-resource-name>, "error out"=w1759:errorcluster)  [unwired: 9 in]
        n1617 = VISA Read(VISA resource name=w1750, byte count=u32 2 ("byte count (0)")) -> (read buffer=w1758:string)  [unwired: 1 in, 3 out]
        n1618 = String Subset(string=w1758, offset (0)=0, length (rest)=2 ("length (rest)")) -> (substring=w1757:string)
        n1619 = Match Pattern(string=w1757, regular expression="<>") -> (offset past match=w1754:i32)  [unwired: 1 in, 3 out]
        n1620 = Greater Or Equal?(x=w1754, y=0) -> (x >= y?=w1749:bool)
        n1621 = case shown="True" w1749 {
          tunnel: w1750 -> [_ w1768]
          tunnel: w1759 -> [_ w1767]
          frame False {
          }
          frame True {
            n1622 = VISA Read(VISA resource name=w1768, byte count=u32 32 ("byte count (0)"), error in (no error)=w1767) -> (read buffer=w1766:string)  [unwired: 3 out]
            n1623 = String Subset(string=w1766, offset (0)=0, length (rest)=8 ("length (rest)")) -> (substring=w1770:string)
            n1624 = String Subset(string=w1766, offset (0)=8, length (rest)=8 ("length (rest)")) -> (substring=w1771:string)
            n1625 = Decimal String To Number(string=w1771) -> (number=w1778:i32)  [unwired: 2 in, 1 out]
            n1626 = Decimal String To Number(string=w1770) -> (number=w1774:i32)  [unwired: 2 in, 1 out]
            n1627 = Divide(x=w1778, y=10000) -> ()  [unwired: 1 out]
            n1628 = Divide(x=w1774, y=1000000) -> ()  [unwired: 1 out]
          }
        }
        n1629 = local read "Quit"() -> (w1747:bool)
      }
    }
    frame Enabled {
    }
  }
  n1630 = Tick Count (ms)() -> (millisecond timer value=w4:u32)
  n1631 = while {
    shift-right: [w1824] -> _
    shift-left: w6 -> [w1828]
    shift-right: [w1823] -> _
    shift-left: w5 -> [w1827]
    shift-right: [w1822] -> _
    shift-left: w6 -> [w1826]
    shift-right: [w1821] -> _
    shift-left: w5 -> [w1825]
    shift-right: [w1819] -> _
    shift-left: w4 -> [w1820]
    shift-right: [w1816] -> _
    shift-left: w3 -> [w1817]
    shift-right: [w1815] -> _
    shift-left: w3 -> [w1818]
    shift-right: [w1808] -> _
    shift-left: w3 -> [w1814]
    shift-right: [w1807] -> _
    shift-left: w3 -> [w1813]
    shift-right: [w1806] -> _
    shift-left: w3 -> [w1812]
    shift-right: [w1805] -> _
    shift-left: w3 -> [w1811]
    shift-right: [w1804] -> _
    shift-left: w3 -> [w1810]
    shift-right: [w1803] -> _
    shift-left: w3 -> [w1809]
    shift-right: [w1802] -> _
    shift-left: w3 -> [w1796]
    shift-right: [w1801] -> _
    shift-left: w3 -> [w1795]
    shift-right: [w1800] -> _
    shift-left: w3 -> [w1794]
    shift-right: [w1799] -> _
    shift-left: w3 -> [w1793]
    shift-right: [w1798] -> _
    shift-left: w3 -> [w1792]
    shift-right: [w1797] -> _
    shift-left: w3 -> [w1791]
    shift-right: [w1782] -> _
    shift-left: w3 -> [w1785]
    shift-right: [w1781] -> _
    shift-left: w3 -> [w1784]
    shift-right: [w1780] -> _
    shift-left: w3 -> [w1783]
    stop <- w1830 stop-if-true
    n1632 = local read "Read UNO"() -> (w1789:string)
    n1633 = local read "Error  2"() -> (w1829:errorcluster)
    n1634 = String Length(string=w1789) -> (length=w1788:i32)
    n1635 = call <vilib>:"Trim Whitespace.vi"("string"=w1789) -> ("trimmed string"=w1790:string)  [unwired: 1 in]
    n1636 = Greater Or Equal?(x=w1788, y=23) -> (x >= y?=w1786:bool)
    n1637 = case shown="No Error" w1829 {
      tunnel: w1828 -> [w1876 w1972]
      tunnel: w1827 -> [w1875 w1971]
      tunnel: w1826 -> [w1874 w1970]
      tunnel: w1825 -> [w1873 w1969]
      tunnel: [w1872 w1972] -> w1824
      tunnel: [w1871 w1971] -> w1823
      tunnel: [w1870 w1970] -> w1822
      tunnel: [w1869 w1969] -> w1821
      tunnel: w1820 -> [w1868 w1968]
      tunnel: [w1867 w1968] -> w1819
      tunnel: w1817 -> [w1866 w1967]
      tunnel: w1818 -> [w1865 w1966]
      tunnel: [w1864 w1967] -> w1816
      tunnel: [w1863 w1966] -> w1815
      tunnel: w1814 -> [w1862 w1965]
      tunnel: w1813 -> [w1861 w1964]
      tunnel: w1812 -> [w1860 w1963]
      tunnel: w1811 -> [w1859 w1962]
      tunnel: w1810 -> [w1858 w1961]
      tunnel: w1809 -> [w1857 w1960]
      tunnel: [w1856 w1965] -> w1808
      tunnel: [w1855 w1964] -> w1807
      tunnel: [w1854 w1963] -> w1806
      tunnel: [w1853 w1962] -> w1805
      tunnel: [w1852 w1961] -> w1804
      tunnel: [w1851 w1960] -> w1803
      tunnel: w1796 -> [w1850 w1959]
      tunnel: [w1849 w1959] -> w1802
      tunnel: [w1848 w1955] -> w1801
      tunnel: [w1847 w1954] -> w1800
      tunnel: [w1846 w1958] -> w1799
      tunnel: [w1845 w1957] -> w1798
      tunnel: [w1844 w1956] -> w1797
      tunnel: w1795 -> [w1843 w1958]
      tunnel: w1794 -> [w1842 w1957]
      tunnel: w1793 -> [w1841 w1956]
      tunnel: w1792 -> [w1840 w1955]
      tunnel: w1791 -> [w1839 w1954]
      tunnel: w1790 -> [w1838 _]
      tunnel: w1786 -> [w1837 _]
      tunnel: w1785 -> [w1836 w1953]
      tunnel: w1784 -> [w1835 w1952]
      tunnel: w1783 -> [w1834 w1951]
      tunnel: [w1833 w1953] -> w1782
      tunnel: [w1832 w1952] -> w1781
      tunnel: [w1831 w1951] -> w1780
      frame No Error {
        n1638 = case shown="True" w1837 {
          tunnel: w1876 -> [w1892 w1944]
          tunnel: w1875 -> [w1891 w1943]
          tunnel: w1874 -> [w1890 w1942]
          tunnel: w1873 -> [w1889 w1941]
          tunnel: [w1892 w1940] -> w1872
          tunnel: [w1891 w1939] -> w1871
          tunnel: [w1890 w1938] -> w1870
          tunnel: [w1889 w1937] -> w1869
          tunnel: w1868 -> [w1888 w1935]
          tunnel: [w1888 w1934] -> w1867
          tunnel: w1866 -> [w1887 w1933]
          tunnel: w1865 -> [w1886 w1932]
          tunnel: [w1887 w1931] -> w1864
          tunnel: [w1886 w1930] -> w1863
          tunnel: w1862 -> [w1885 w1929]
          tunnel: w1861 -> [w1884 w1928]
          tunnel: w1860 -> [w1883 w1927]
          tunnel: w1859 -> [w1882 w1926]
          tunnel: w1858 -> [w1881 w1925]
          tunnel: w1857 -> [w1880 w1924]
          tunnel: [w1885 w1923] -> w1856
          tunnel: [w1884 w1922] -> w1855
          tunnel: [w1883 w1921] -> w1854
          tunnel: [w1882 w1920] -> w1853
          tunnel: [w1881 w1919] -> w1852
          tunnel: [w1880 w1918] -> w1851
          tunnel: w1850 -> [w1898 w1917]
          tunnel: [w1898 w1916] -> w1849
          tunnel: [w1895 w1915] -> w1848
          tunnel: [w1894 w1914] -> w1847
          tunnel: [w1897 w1913] -> w1846
          tunnel: [w1893 w1912] -> w1845
          tunnel: [w1896 w1911] -> w1844
          tunnel: w1843 -> [w1897 w1910]
          tunnel: w1842 -> [w1896 w1909]
          tunnel: w1841 -> [w1895 w1908]
          tunnel: w1840 -> [w1894 w1907]
          tunnel: w1839 -> [w1893 w1906]
          tunnel: w1838 -> [_ w1905]
          tunnel: w1836 -> [w1879 w1904]
          tunnel: w1835 -> [w1878 w1903]
          tunnel: w1834 -> [w1877 w1902]
          tunnel: [w1879 w1901] -> w1833
          tunnel: [w1878 w1900] -> w1832
          tunnel: [w1877 w1899] -> w1831
          frame False {
          }
          frame True {
            n1639 = Tick Count (ms)() -> (millisecond timer value=w1936:u32)
            n1640 = String To Byte Array(string=w1905) -> (unsigned byte array=w1949:u8[])
            n1641 = Array Size(array=w1949) -> (size(s)=w1948:i32)
            n1642 = formula code="// --- INTERNAL VARIABLE DECLARATIONS ---\nint i = 0;\nint k = 0;\nint start_idx = -1;\nint end_idx = -1;\nint phase = 0;\nint sign0 = 1;\nint sign1 = 1;\nint ch0_val = 0;   \nint ch1_val = 0;   \nfloat ch0_raw = 0.0;\nfloat ch1_raw = 0.0;\nfloat temp0 = 0.0;\nfloat temp1 = 0.0;\nfloat ch0_clean = 0.0;\nfloat ch1_clean = 0.0;\n\nint valid_samples = 0; // FIX: Track if we actually parsed new data this window\nfloat max_allowed_bits = 8388607.0; // FIX: Change this to match your ADC max value\n\n// Temporal intermediate variables for calculation smoothing\nfloat raw_p2p_v = 0.0;\nfloat raw_friction = 0.0;\nfloat raw_cof = 0.0;\n\n// Temporal intermediate variables for Piezo voltage translations\nfloat piezo_min_v = 0.0;\nfloat piezo_max_v = 0.0;\n\n// Initialize output variables to current shift register states right away\nout_LVDT_Min_V = in_LVDT_Min_V;\nout_LVDT_Max_V = in_LVDT_Max_V;\nout_LVDT_P2P_V = in_LVDT_P2P_V;\nout_Piezo_P2P = in_Piezo_P2P;\nout_Friction_N = in_Friction_N;\nout_COF = in_COF;\nwindow_ready = 0;\n\n// --- STEP 1: PARSE EVERY STRING IN THE BYTE ARRAY ---\nif (array_size > 2) {\n    for (i = 0; i < array_size - 1; i++) {\n        if (raw_bytes[i] == 42) { // '*' character detected\n            start_idx = i;\n        }\n        \n        // Match standard delimiter sequence \";&\" or end window character\n        if (raw_bytes[i] == 59 && raw_bytes[i+1] == 38 && start_idx != -1) { \n            end_idx = i;\n            ch0_val = 0;\n            ch1_val = 0;\n            sign0 = 1;\n            sign1 = 1;\n            phase = 0; \n\n            for (k = start_idx + 1; k < end_idx; k++) {\n                if (raw_bytes[k] == 45) { // '-' sign\n                    if (phase == 0) sign0 = -1;\n                    else sign1 = -1;\n                }\n                else if (raw_bytes[k] == 43) { // '+' sign\n                    if (phase == 0) sign0 = 1;\n                    else sign1 = 1;\n                }\n                else if (raw_bytes[k] == 59) { // ';' delimiter\n                    phase = 1; \n                }\n                else if (raw_bytes[k] >= 48 && raw_bytes[k] <= 57) { // Numeric ASCII digits\n                    if (phase == 0) {\n                        ch0_val = (ch0_val * 10) + (raw_bytes[k] - 48);\n                    } else {\n                        ch1_val = (ch1_val * 10) + (raw_bytes[k] - 48);\n                    }\n                }\n            }\n\n            // Implicit type conversion\n            ch0_raw = ch0_val * sign0 * 1.0;\n            ch1_raw = ch1_val * sign1 * 1.0;\n\n            // FIX: Sanity check / Hard-clamping to catch sudden massive ASCII noise spikes\n            if (ch0_raw > max_allowed_bits)  ch0_raw = max_allowed_bits;\n            if (ch0_raw < -max_allowed_bits) ch0_raw = -max_allowed_bits;\n            if (ch1_raw > max_allowed_bits)  ch1_raw = max_allowed_bits;\n            if (ch1_raw < -max_allowed_bits) ch1_raw = -max_allowed_bits;\n\n            // --- STEP 2: 3-SAMPLE MEDIAN FILTER ---\n            m0_2 = m0_1; m0_1 = m0_0; m0_0 = ch0_raw;\n            float s0_0 = m0_0; float s0_1 = m0_1; float s0_2 = m0_2;\n            if (s0_0 > s0_1) { temp0 = s0_0; s0_0 = s0_1; s0_1 = temp0; }\n            if (s0_1 > s0_2) { temp0 = s0_1; s0_1 = s0_2; s0_2 = temp0; }\n            if (s0_0 > s0_1) { temp0 = s0_0; s0_0 = s0_1; s0_1 = temp0; }\n            ch0_clean = s0_1;\n\n            m1_2 = m1_1; m1_1 = m1_0; m1_0 = ch1_raw;\n            float s1_0 = m1_0; float s1_1 = m1_1; float s1_2 = m1_2;\n            if (s1_0 > s1_1) { temp1 = s1_0; s1_0 = s1_1; s1_1 = temp1; }\n            if (s1_1 > s1_2) { temp1 = s1_1; s1_1 = s1_2; s1_2 = temp1; }\n            if (s1_0 > s1_1) { temp1 = s1_0; s1_0 = s1_1; s1_1 = temp1; }\n            ch1_clean = s1_1;\n\n            // --- STEP 3: EXPONENTIAL FILTER (STREAM LEVEL) ---\n            if (ch0_filt == 0.0) ch0_filt = ch0_clean;\n            if (ch1_filt == 0.0) ch1_filt = ch1_clean;\n\n            ch0_filt = ch0_filt + (ch0_clean - ch0_filt) * 0.125;\n            ch1_filt = ch1_filt + (ch1_clean - ch1_filt) * 0.125;\n\n            // --- STEP 4: MIN/MAX WINDOW CONTINUOUS ACCUMULATION ---\n            if (ch0_filt > max_ch0) max_ch0 = ch0_filt;\n            if (ch0_filt < min_ch0) min_ch0 = ch0_filt;\n            if (ch1_filt > max_ch1) max_ch1 = ch1_filt;\n            if (ch1_filt < min_ch1) min_ch1 = ch1_filt;\n\n            valid_samples++; // FIX: Successfully parsed and accumulated a clean point\n            start_idx = -1; \n        }\n    }\n}\n\n// --- STEP 5: WINDOW EVALUATION ENGINE ---\n// FIX: Condition updated to verify that valid samples exist for both channels\nif (((current_time_ms - start_time_ms) >= 50) && (valid_samples > 0) && (min_ch0 < 9000000.0) && (min_ch1 < 9000000.0)) {\n    window_ready = 1;\n\n    // Linear Bit-to-Voltage Transformations (LVDT - Channel 0)\n    out_LVDT_Min_V = (min_ch0 * VREF) / 8388607.0;\n    out_LVDT_Max_V = (max_ch0 * VREF) / 8388607.0;\n    raw_p2p_v = out_LVDT_Max_V - out_LVDT_Min_V;\n\n    // Linear Bit-to-Voltage Transformations (Piezo - Channel 1)\n    piezo_min_v = (min_ch1 * VREF) / 8388607.0;\n    piezo_max_v = (max_ch1 * VREF) / 8388607.0;\n    \n    // Assign Peak-to-Peak Voltage directly to output indicator (Matches Python logic)\n    out_Piezo_P2P = piezo_max_v - piezo_min_v;\n    \n    // Force scaling calculations using Voltage delta * Newtons/Volt Factor\n    raw_friction = out_Piezo_P2P * PIEZO_CAL_FACTOR + 0.44528;\n    raw_cof = raw_friction / NORMAL_FORCE;\n\n    // --- STEP 6: OUTPUT METRIC SMOOTHING (Low-Pass Filter Alpha = 0.05) ---\n    // Seed initial historical metrics if first loop iteration\n    if (hist_LVDT_P2P == 0.0) hist_LVDT_P2P = raw_p2p_v;\n    if (hist_Friction == 0.0) hist_Friction = raw_friction;\n    if (hist_COF == 0.0)      hist_COF = raw_cof;\n\n    // Apply exponential output dampening\n    hist_LVDT_P2P = hist_LVDT_P2P + (raw_p2p_v - hist_LVDT_P2P) * 0.05;\n    hist_Friction = hist_Friction + (raw_friction - hist_Friction) * 0.05; // Note: Can drop to 0.02 for more aggressive damping\n    hist_COF      = hist_COF + (raw_cof - hist_COF) * 0.05;\n\n    // Direct smoothed parameters out to UI Indicators\n    out_LVDT_P2P_V = hist_LVDT_P2P;\n    out_Friction_N = hist_Friction;\n    out_COF        = hist_COF;\n\n    // Reset tracking targets to extreme boundaries safely\n    min_ch0 = 9999999.0;\n    max_ch0 = -9999999.0;\n    min_ch1 = 9999999.0;\n    max_ch1 = -9999999.0;\n\n    valid_samples = 0; // FIX: Reset counter for next time frame\n    start_time_ms = current_time_ms;\n}"("raw_bytes"=w1949, "array_size"=w1948, "VREF"="VREF", "PIEZO_CAL_FACTOR"="PIEZO_CAL_FACTOR", "NORMAL_FORCE"="NORMAL_FORCE", "min_ch0"=w1944, "max_ch0"=w1943, "min_ch1"=w1942, "max_ch1"=w1941, "current_time_ms"=w1936, "start_time_ms"=w1935, "ch0_filt"=w1933, "ch1_filt"=w1932, "m0_0"=w1929, "m0_1"=w1928, "m0_2"=w1927, "m1_0"=w1926, "m1_1"=w1925, "m1_2"=w1924, "in_LVDT_Min_V"=w1917, "in_LVDT_Max_V"=w1910, "in_LVDT_P2P_V"=w1909, "in_Piezo_P2P"=w1908, "in_Friction_N"=w1907, "in_COF"=w1906, "hist_LVDT_P2P"=w1904, "hist_Friction"=w1903, "hist_COF"=w1902) -> ("window_ready"=→"Valid_data":dbl, "out_LVDT_Min_V"=w1916:dbl, "out_LVDT_Max_V"=w1915:dbl, "out_LVDT_P2P_V"=w1914:dbl, "out_Piezo_P2P"=w1913:dbl, "out_Friction_N"=w1912:dbl, "out_COF"=w1911:dbl, "min_ch0"=w1940:dbl, "max_ch0"=w1939:dbl, "min_ch1"=w1938:dbl, "max_ch1"=w1937:dbl, "start_time_ms"=w1934:u32, "ch0_filt"=w1931:dbl, "ch1_filt"=w1930:dbl, "m0_0"=w1923:dbl, "m0_1"=w1922:dbl, "m0_2"=w1921:dbl, "m1_0"=w1920:dbl, "m1_1"=w1919:dbl, "m1_2"=w1918:dbl, "hist_LVDT_P2P"=w1901:dbl, "hist_Friction"=w1900:dbl, "hist_COF"=w1899:dbl)
            "LVDT MIN" <- w1916
            "LVDT MAX" <- w1915
            "LVDT Peak" <- w1914
            "pizo raw" <- w1913
            "cof" <- w1911
            "Frictioin Force Raw" <- w1912
          }
        }
      }
      frame Error {
      }
    }
    n1643 = local read "Quit"() -> (w1830:bool)
  }
  n1644 = disable-structure shown="Disabled" {
    disable-tunnel: errorcluster {"status"=TRUE, "code"=0, "source"="Init"} ("error IO") -> [w1975 _]
    disable-tunnel: [w1973 _] -> w45
    frame Disabled {
      n1645 = while {
        shift-right: [w1991] -> w1977
        shift-left: _ -> [w1982]
        shift-right: [w1990] -> w1976
        shift-left: w1975 -> [w1984]
        tunnel: [w1979] -> w1973
        tunnel: [w1989] -> _
        i -> [w1989]
        stop <- w1979 stop-if-true
        n1646 = local read "Port 1a"() -> (w1985:bool)
        n1647 = local read "Port 3"() -> (w1986:bool)
        n1648 = local read "Com Port 1"() -> (w1983:refnum<visa-resource-name>)
        n1649 = Or(x=w1986, y=w1985) -> (x .or. y?=w1988:bool)
        n1650 = Unbundle(w1984) -> ("status"=→"Port 3":bool)  [unwired: 2 out]
        n1651 = Not Equal?(x=w1983, y=w1982) -> (x != y?=w1980:bool)
        n1652 = case shown="True" w1988 {
          frame False {
            w1994 = TRUE ("Visible")
            n1653 = property on="Port 1a" class="Bool (strict)"("Visible"=w1994) -> ()  [unwired: 2 in, 2 out]
            n1654 = property on="Port 3" class="Bool (strict)"("Visible"=w1994) -> ()  [unwired: 2 in, 2 out]
          }
          frame True {
            w1995 = TRUE ("Visible")
            n1655 = property on="Port 1a" class="Bool (strict)"("Visible"=w1995) -> ()  [unwired: 2 in, 2 out]
            n1656 = property on="Port 3" class="Bool (strict)"("Visible"=w1995) -> ()  [unwired: 2 in, 2 out]
          }
        }
        n1657 = Wait (ms)(milliseconds to wait=u32 40) -> ()  [unwired: 1 out]
        n1658 = case shown="True" w1980 {
          tunnel: [w1992 errorcluster {"status"=TRUE, "code"=0, "source"="Init"} ("error out")] -> w1981
          tunnel: w1984 -> [w1992 _]
          frame False {
          }
          frame True {
          }
        }
        n1659 = case shown="Error" w1981 {
          selector: w1981 -> [w2002 w2020]
          tunnel: [w2005 w2024] -> w1991
          tunnel: [w2004 w2018] -> w1990
          tunnel: w1982 -> [w2003 w2022]
          frame No Error {
            n1660 = property class="Instr"(reference=w2003, error in=w2002) -> (reference out=w2000:refnum<visa-resource-name>, error out=w2001:errorcluster, "Serial Settings:Number of Bytes at Serial Port"=w1997:u32)
            n1661 = Greater?(x=w1997, y=u32 5) -> (0:w1996:bool)
            n1662 = Not(x=w1996) -> (.not. x?=→"Port 1a":bool)
            n1663 = while {
              tunnel: [w2013] -> w2004
              tunnel: [w2012] -> w2005
              tunnel: w2001 -> [w2011]
              tunnel: w2000 -> [w2010]
              stop <- TRUE stop-if-true
              n1664 = property class="Instr" props=["Serial Settings:Number of Bytes at Serial Port"](reference=w2010, error in=w2011) -> (reference out=w2015:refnum<visa-resource-name>, error out=w2014:errorcluster)  [unwired: 1 out]
              n1665 = VISA Read(VISA resource name=w2015, byte count=u32 50, error in (no error)=w2014) -> (VISA resource name out=w2012:refnum<visa-resource-name>, read buffer=w2007:string, error out=w2013:errorcluster)  [unwired: 1 out]
              n1666 = Wait (ms)(milliseconds to wait=u32 5) -> ()  [unwired: 1 out]
            }
          }
          frame Error {
            w2030 = u16 0 items=["None", "XON/XOFF", "RTS/CTS", "XON/XOFF & RTS/CTS", "DTR/DSR", "XON/XOFF & DTR/DSR"] ("flow control (0:none)  2")
            w2028 = u16 10 items=["1.0"=10, "1.5"=15, "2.0"=20] ("stop bits 2")
            w2026 = u16 0 items=["None", "Odd", "Even", "Mark", "Space"] ("parity 2")
            w2027 = u32 10000  # timeout (10sec)
            n1667 = VISA Close(VISA resource name=w2022, error in (no error)=w2020) -> (error out=w2023:errorcluster)
            n1668 = local write "Port 1a"(FALSE ("Port 1a")) -> ()
            n1669 = local read "Com Port 1"() -> (w2017:refnum<visa-resource-name>)
            n1670 = call <vilib>:"Clear Errors.vi"("error in (no error)"=w2023) -> ("error out"=w2021:errorcluster)  [unwired: 5 in, 1 out]
            n1671 = call-poly "VISA Configure Serial Port"("VISA resource name"=w2017, "timeout (10sec)"=w2027, "baud rate (9600)"=u32 250000 ("baud rate  2"), "data bits (8)"=u16 8 ("data bits  2"), "parity (0:none)"=w2026, "error in (no error)"=w2021, "stop bits (10: 1 bit)"=w2028, "flow control (0:none)"=w2030) -> ("VISA resource name out"=w2031:refnum<visa-resource-name>, "error out"=w2032:errorcluster)  [unwired: 6 in]
            n1672 = flat-sequence {
              tunnel: w2031 -> [w2034]
              tunnel: w2032 -> [w2033]
              tunnel: [w2034] -> w2024
              tunnel: [w2033] -> w2018
              frame #0 {
                n1673 = Wait (ms)(milliseconds to wait=u32 50) -> ()  [unwired: 1 out]
              }
            }
            "Residual Uno" <- ""
          }
        }
        n1674 = local read "Quit"() -> (w1979:bool)
        "Error Uno" <- w1984
      }
      n1675 = VISA Close(VISA resource name=w1977, error in (no error)=w1976) -> (error out=w1974:errorcluster)
      n1676 = call <vilib>:"Clear Errors.vi"("error in (no error)"=w1974) -> ()  [unwired: 5 in, 2 out]
    }
    frame Enabled {
    }
  }
  n1677 = while {
    stop <- w2045 stop-if-true
    # "V0OLTAGE TO STROKE (peice vise calibration)"
    n1678 = local read "LVDT MIN"() -> (w2037:dbl)
    n1679 = local read "LVDT Peak"() -> (w2036:dbl)
    n1680 = Wait (ms)(milliseconds to wait=u32 10) -> ()  [unwired: 1 out]
    n1681 = formula code="// Dynamic Parameterized Linear Interpolation Node\n// Inputs: vpp_val, voltages (Array), distances (Array)\n// Outputs: stroke\n\nint i = 0;\nint segments = 11; // 12 points make 11 interpolation segments\n\n// 1. Lower Boundary Clamp\nif (vpp_val <= voltages[0]) {\n    stroke = distances[0];\n}\n// 2. Upper Boundary Clamp\nelse if (vpp_val >= voltages[segments]) {\n    stroke = distances[segments];\n}\n// 3. Dynamic Segment Search Loop\nelse {\n    stroke = distances[0]; // Fallback baseline\n    for (i = 0; i < segments; i++) {\n        if (vpp_val >= voltages[i] && vpp_val <= voltages[i+1]) {\n            // Standard linear interpolation formula using array lookups\n            stroke = distances[i] + (vpp_val - voltages[i]) * (distances[i+1] - distances[i]) / (voltages[i+1] - voltages[i]);\n            break; // Segment found, safely exit the loop\n        }\n    }\n}"("vpp_val"=w2036, "voltages"="calibration values", "distances"="STROKE") -> ("stroke"=→"LVDT STROKE":dbl)
    n1682 = local read "Calibration Tare Value"() -> (w2041:dbl)
    n1683 = local read "Calibration Tare"() -> (w2039:bool)
    n1684 = Subtract(x=w2037, y=w2041) -> (x-y=→"LVDT STROKE  Calibration":dbl)